vi "Velociprobe_Nanopositioner_Control_RT 2.vi"() -> ()   [LabVIEW 2015] (continued)
        n12 = invoke on="Waveform Graph 2" class="WFGraph (strict)" method="Reinit To Default"() -> (error out=w50:errorcluster)  [unwired: 3 in, 2 out]
        n13 = xnode "Read/Write Control"("FPGA VI Reference In"=w42, "error in"=w41) -> ("FPGA VI Reference Out"=w40:refnum<k20>, "error out"=w39:errorcluster, "error out (FPGA)"=w57:errorcluster)
        n14 = Merge Errors "Merge Errors"(w39, w57, w50) -> (w38:errorcluster)
      }
      frame "Update Controller Info" {
        w294 = dbl[] [1.0, 2.0, 4.0, 5.0]  # Index_soscoeff_zz1
        w133 = dbl[] [1.0, 2.0, 4.0, 5.0]  # Index_soscoeff_yz1
        w154 = dbl[] [1.0, 2.0, 4.0, 5.0]  # Index_soscoeff_xz1
        w185 = dbl[] [1.0, 2.0, 4.0, 5.0]  # Index_soscoeff_zy1
        w315 = dbl[] [1.0, 2.0, 4.0, 5.0]  # Index_soscoeff_yy1
        w206 = dbl[] [1.0, 2.0, 4.0, 5.0]  # Index_soscoeff_xy1
        w232 = dbl[] [1.0, 2.0, 4.0, 5.0]  # Index_soscoeff_zx1
        w341 = dbl[] [1.0, 2.0, 4.0, 5.0]  # Index_soscoeff_xx1
        w258 = dbl[] [1.0, 2.0, 4.0, 5.0]  # Index_soscoeff_yx1
        w114 = "%.10f"  # format (%.3f)
        w122 = "%.10f"  # format (%.3f)
        w135 = "%.10f"  # format (%.3f)
        w143 = "%.10f"  # format (%.3f)
        w166 = "%.10f"  # format (%.3f)
        w174 = "%.10f"  # format (%.3f)
        w187 = "%.10f"  # format (%.3f)
        w195 = "%.10f"  # format (%.3f)
        w213 = "%.10f"  # format (%.3f)
        w221 = "%.10f"  # format (%.3f)
        w239 = "%.10f"  # format (%.3f)
        w247 = "%.10f"  # format (%.3f)
        w275 = "%.10f"  # format (%.3f)
        w283 = "%.10f"  # format (%.3f)
        w296 = "%.10f"  # format (%.3f)
        w304 = "%.10f"  # format (%.3f)
        w105 = fxp<+/-,42,9> 0.0 ("fixed-point type")
        w317 = "%.10f"  # format (%.3f)
        w104 = fxp<+/-,64,9> 0.0 ("fixed-point type")
        w330 = "%.10f"  # format (%.3f)
        w348 = 40000000.0  # FPGA Clock Rate (Hz)
        w81 = 1
        n15 = local read "sos gain SF Controller yy1c"() -> (w269:fxp<+/-,42,9>)
        n16 = local read "sos gain SF Controller yz1c"() -> (w90:fxp<+/-,42,9>)
        n17 = local read "sos gain SF Controller yx1c"() -> (w236:fxp<+/-,42,9>)
        n18 = local read "sos gain SF Controller xy1c"() -> (w159:fxp<+/-,42,9>)
        n19 = local read "sos gain SF Controller zy1c"() -> (w164:fxp<+/-,42,9>)
        n20 = local read "sos gain SF Controller xz1c"() -> (w106:fxp<+/-,42,9>)
        n21 = local read "sos gain SF Controller xx1c"() -> (w319:fxp<+/-,42,9>)
        n22 = local read "sos gain SF Controller zz1c"() -> (w267:fxp<+/-,42,9>)
        n23 = local read "sos gain SF Controller zx1c"() -> (w211:fxp<+/-,42,9>)
        n24 = local read "-a01(2) yy1c"() -> (w273:fxp<+/-,64,9>[])
        n25 = local read "-a02(2) yy1c"() -> (w272:fxp<+/-,64,9>[])
        n26 = local read "-a01(2) yz1c"() -> (w111:fxp<+/-,64,9>[])
        n27 = local read "-a02(2) yz1c"() -> (w112:fxp<+/-,64,9>[])
        n28 = local read "-a01(2) yx1c"() -> (w237:fxp<+/-,64,9>[])
        n29 = local read "-a02(2) yx1c"() -> (w233:fxp<+/-,64,9>[])
        n30 = local read "-a01(2) xy1c"() -> (w155:fxp<+/-,64,9>[])
        n31 = local read "-a02(2) xy1c"() -> (w156:fxp<+/-,64,9>[])
        n32 = local read "-a01(2) zy1c"() -> (w160:fxp<+/-,64,9>[])
        n33 = local read "-a02(2) zy1c"() -> (w161:fxp<+/-,64,9>[])
        n34 = local read "-a01(2) xz1c"() -> (w110:fxp<+/-,64,9>[])
        n35 = local read "-a02(2) xz1c"() -> (w109:fxp<+/-,64,9>[])
        n36 = local read "-a01(2) xx1c"() -> (w328:fxp<+/-,64,9>[])
        n37 = local read "-a02(2) xx1c"() -> (w327:fxp<+/-,64,9>[])
        n38 = local read "-a01(2) zz1c"() -> (w268:fxp<+/-,64,9>[])
        n39 = local read "-a02(2) zz1c"() -> (w264:fxp<+/-,64,9>[])
        n40 = local read "-a01(2) zx1c"() -> (w207:fxp<+/-,64,9>[])
        n41 = local read "-a02(2) zx1c"() -> (w208:fxp<+/-,64,9>[])
        n42 = local read "b01(2) yy1c"() -> (w271:fxp<+/-,64,9>[])
        n43 = local read "b02(2) yy1c"() -> (w270:fxp<+/-,64,9>[])
        n44 = local read "b01(2) yz1c"() -> (w76:fxp<+/-,64,9>[])
        n45 = local read "b02(2) yz1c"() -> (w75:fxp<+/-,64,9>[])
        n46 = local read "b01(2) yx1c"() -> (w234:fxp<+/-,64,9>[])
        n47 = local read "b02(2) yx1c"() -> (w235:fxp<+/-,64,9>[])
        n48 = local read "b01(2) xy1c"() -> (w157:fxp<+/-,64,9>[])
        n49 = local read "b02(2) xy1c"() -> (w158:fxp<+/-,64,9>[])
        n50 = local read "b01(2) zy1c"() -> (w162:fxp<+/-,64,9>[])
        n51 = local read "b02(2) zy1c"() -> (w163:fxp<+/-,64,9>[])
        n52 = local read "b01(2) xz1c"() -> (w108:fxp<+/-,64,9>[])
        n53 = local read "b02(2) xz1c"() -> (w107:fxp<+/-,64,9>[])
        n54 = local read "b01(2) xx1c"() -> (w326:fxp<+/-,64,9>[])
        n55 = local read "b02(2) xx1c"() -> (w325:fxp<+/-,64,9>[])
        n56 = local read "b01(2) zz1c"() -> (w265:fxp<+/-,64,9>[])
        n57 = local read "b02(2) zz1c"() -> (w266:fxp<+/-,64,9>[])
        n58 = local read "b01(2) zx1c"() -> (w209:fxp<+/-,64,9>[])
        n59 = local read "b02(2) zx1c"() -> (w210:fxp<+/-,64,9>[])
        n60 = Or(x="Optics Z Reset", y="Reset All") -> (x .or. y?=w103:bool)
        n61 = Or(x="Sample Z Reset", y="Reset All") -> (x .or. y?=w100:bool)
        n62 = Or(x="Optics X Reset", y="Reset All") -> (x .or. y?=w262:bool)
        n63 = Or(x="Optics Y Reset", y="Reset All") -> (x .or. y?=w260:bool)
        n64 = Or(x="Sample X Reset", y="Reset All") -> (x .or. y?=w102:bool)
        n65 = Or(x="Sample Y Reset", y="Reset All") -> (x .or. y?=w101:bool)
        n66 = call-poly <vilib>:"Read Delimited Spreadsheet.vi"("file path (dialog if empty)"="file path soscoeff_xx1", "format (%.3f)"=w330) -> ("all rows"=w329:dbl[][])  [unwired: 8 in, 5 out]
        n67 = call-poly <vilib>:"Read Delimited Spreadsheet.vi"("file path (dialog if empty)"="file path soscoeff_zy1", "format (%.3f)"=w174) -> ("all rows"=w173:dbl[][])  [unwired: 8 in, 5 out]
        n68 = call-poly <vilib>:"Read Delimited Spreadsheet.vi"("file path (dialog if empty)"="file path soscoeff_xy1", "format (%.3f)"=w195) -> ("all rows"=w194:dbl[][])  [unwired: 8 in, 5 out]
        n69 = call-poly <vilib>:"Read Delimited Spreadsheet.vi"("file path (dialog if empty)"="file path soscoeff_zx1", "format (%.3f)"=w221) -> ("all rows"=w220:dbl[][])  [unwired: 8 in, 5 out]
        n70 = call-poly <vilib>:"Read Delimited Spreadsheet.vi"("file path (dialog if empty)"="file path soscoeff_xz1", "format (%.3f)"=w143) -> ("all rows"=w142:dbl[][])  [unwired: 8 in, 5 out]
        n71 = call-poly <vilib>:"Read Delimited Spreadsheet.vi"("file path (dialog if empty)"="file path soscoeff_yx1", "format (%.3f)"=w247) -> ("all rows"=w246:dbl[][])  [unwired: 8 in, 5 out]
        n72 = call-poly <vilib>:"Read Delimited Spreadsheet.vi"("file path (dialog if empty)"="file path soscoeff_yy1", "format (%.3f)"=w304) -> ("all rows"=w303:dbl[][])  [unwired: 8 in, 5 out]
        n73 = call-poly <vilib>:"Read Delimited Spreadsheet.vi"("file path (dialog if empty)"="file path soscoeff_yz1", "format (%.3f)"=w122) -> ("all rows"=w121:dbl[][])  [unwired: 8 in, 5 out]
        n74 = call-poly <vilib>:"Read Delimited Spreadsheet.vi"("file path (dialog if empty)"="file path soscoeff_zz1", "format (%.3f)"=w283) -> ("all rows"=w282:dbl[][])  [unwired: 8 in, 5 out]
        n75 = Transpose 2D Array(2D array=w329) -> (transposed array=w340:dbl[][])
        n76 = Transpose 2D Array(2D array=w173) -> (transposed array=w184:dbl[][])
        n77 = Transpose 2D Array(2D array=w194) -> (transposed array=w205:dbl[][])
        n78 = Transpose 2D Array(2D array=w220) -> (transposed array=w231:dbl[][])
        n79 = Transpose 2D Array(2D array=w142) -> (transposed array=w153:dbl[][])
        n80 = Transpose 2D Array(2D array=w246) -> (transposed array=w257:dbl[][])
        n81 = Transpose 2D Array(2D array=w303) -> (transposed array=w314:dbl[][])
        n82 = Transpose 2D Array(2D array=w121) -> (transposed array=w132:dbl[][])
        n83 = Transpose 2D Array(2D array=w282) -> (transposed array=w293:dbl[][])
        n84 = call-poly <vilib>:"Read Delimited Spreadsheet.vi"("file path (dialog if empty)"="file path sos gain SF Controller_xx1", "format (%.3f)"=w317) -> ("all rows"=w316:dbl[][])  [unwired: 8 in, 5 out]
        n85 = call-poly <vilib>:"Read Delimited Spreadsheet.vi"("file path (dialog if empty)"="file path sos gain SF Controller_zy1", "format (%.3f)"=w166) -> ("all rows"=w165:dbl[][])  [unwired: 8 in, 5 out]
        n86 = call-poly <vilib>:"Read Delimited Spreadsheet.vi"("file path (dialog if empty)"="file path sos gain SF Controller_xy1", "format (%.3f)"=w187) -> ("all rows"=w186:dbl[][])  [unwired: 8 in, 5 out]
        n87 = call-poly <vilib>:"Read Delimited Spreadsheet.vi"("file path (dialog if empty)"="file path sos gain SF Controller_zx1", "format (%.3f)"=w213) -> ("all rows"=w212:dbl[][])  [unwired: 8 in, 5 out]
        n88 = call-poly <vilib>:"Read Delimited Spreadsheet.vi"("file path (dialog if empty)"="file path sos gain SF Controller_xz1", "format (%.3f)"=w135) -> ("all rows"=w134:dbl[][])  [unwired: 8 in, 5 out]
        n89 = call-poly <vilib>:"Read Delimited Spreadsheet.vi"("file path (dialog if empty)"="file path sos gain SF Controller_yx1", "format (%.3f)"=w239) -> ("all rows"=w238:dbl[][])  [unwired: 8 in, 5 out]
        n90 = call-poly <vilib>:"Read Delimited Spreadsheet.vi"("file path (dialog if empty)"="file path sos gain SF Controller_yy1", "format (%.3f)"=w296) -> ("all rows"=w295:dbl[][])  [unwired: 8 in, 5 out]
        n91 = call-poly <vilib>:"Read Delimited Spreadsheet.vi"("file path (dialog if empty)"="file path sos gain SF Controller_yz1", "format (%.3f)"=w114) -> ("all rows"=w113:dbl[][])  [unwired: 8 in, 5 out]
        n92 = call-poly <vilib>:"Read Delimited Spreadsheet.vi"("file path (dialog if empty)"="file path sos gain SF Controller_zz1", "format (%.3f)"=w275) -> ("all rows"=w274:dbl[][])  [unwired: 8 in, 5 out]
        n93 = xnode "Read/Write Control"("FPGA VI Reference In"=w69, "error in"=w70, "Controller Time Period (uSec)"="Controller Time Period (uSec)", "Controller Output Time Period (uSec)"="Controller Output Time Period (uSec)", "System Loop Type"="System Loop Type", "Controller Output Upper Limit"="Controller Output Upper Limit", "Controller Output Lower Limit"="Controller Output Lower Limit", "X-Stage nm to V Scaling"="X-Stage nm to V Scaling", "X-Stage Scaling Direction"="X-Stage Scaling Direction", "Y-Stage nm to V Scaling"="Y-Stage nm to V Scaling", "Z-Stage nm to V Scaling"="Z-Stage nm to V Scaling", "Plant Output Time Period (uSec)"="Plant Output Time Period (uSec)", "Reset Optics X"=w262, "Reset Optics Y"=w260, "Reset Optics Z"=w103, "Reset Sample X"=w102, "Reset Sample Y"=w101, "Reset Sample Z"=w100, "Optics X Stage Resolution (nm)"="Optics X Stage Resolution (nm)", "Optics Y Stage Resolution (nm)"="Optics Y Stage Resolution (nm)", "Optics Z Stage Resolution (nm)"="Optics Z Stage Resolution (nm)", "Sample X Stage Resolution (nm)"="Sample X Stage Resolution (nm)", "Sample Y Stage Resolution (nm)"="Sample Y Stage Resolution (nm)", "Sample Z Stage Resolution (nm)"="Sample Z Stage Resolution (nm)", "Scaling mV to V"="Scaling mV to V", "-a01(2) xx1"=w328, "-a02(2) xx1"=w327, "b01(2) xx1"=w326, "b02(2) xx1"=w325, "sos gain SF Controller xx1"=w319, "-a01(2) yy1"=w273, "-a02(2) yy1"=w272, "b01(2) yy1"=w271, "b02(2) yy1"=w270, "sos gain SF Controller yy1"=w269, "-a01(2) zz1"=w268, "-a02(2) zz1"=w264, "b01(2) zz1"=w265, "b02(2) zz1"=w266, "sos gain SF Controller zz1"=w267, "-a01(2) yx1"=w237, "-a02(2) yx1"=w233, "b01(2) yx1"=w234, "b02(2) yx1"=w235, "sos gain SF Controller yx1"=w236, "-a01(2) zx1"=w207, "-a02(2) zx1"=w208, "b01(2) zx1"=w209, "b02(2) zx1"=w210, "sos gain SF Controller zx1"=w211, "-a01(2) xy1"=w155, "-a02(2) xy1"=w156, "b01(2) xy1"=w157, "b02(2) xy1"=w158, "sos gain SF Controller xy1"=w159, "-a01(2) zy1"=w160, "-a02(2) zy1"=w161, "b01(2) zy1"=w162, "b02(2) zy1"=w163, "sos gain SF Controller zy1"=w164, "-a01(2) xz1"=w110, "-a02(2) xz1"=w109, "b01(2) xz1"=w108, "b02(2) xz1"=w107, "sos gain SF Controller xz1"=w106, "-a01(2) yz1"=w111, "-a02(2) yz1"=w112, "b01(2) yz1"=w76, "b02(2) yz1"=w75, "sos gain SF Controller yz1"=w90, "Analog Input Time Period (uSec)"="Analog Input Time Period (uSec)", "Optics and or Sample Stage"="Optics and or Sample Stage", "Y-Stage Scaling Direction"="Y-Stage Scaling Direction", "Z-Stage Scaling Direction"="Z-Stage Scaling Direction") -> ("FPGA VI Reference Out"=w68:refnum<k20>, "error out"=w67:errorcluster)
        n94 = for {
          tunnel: w341 -> [w517] mode=indexing
          tunnel: w340 -> [w516]
          tunnel: [w515] -> _ mode=indexing
          shift-right: [w515] -> w332
          shift-left: _ -> [w514]
          shift-left: _ -> [w513]
          shift-left: _ -> [w512]
          tunnel: [w514] -> w333
          tunnel: [w513] -> w334
          tunnel: [w512] -> w335
          n95 = Index Array "Index Array"(array=w516, index (row)=w517) -> (element=w515:dbl[])  [unwired: 1 in]
        }
        n96 = Index Array(array=w316, index (row)=0 ("index (row) 6")) -> (element=w324:dbl[])  [unwired: 1 in]
        n97 = for {
          tunnel: w185 -> [w415] mode=indexing
          tunnel: w184 -> [w414]
          tunnel: [w413] -> _ mode=indexing
          shift-right: [w413] -> w176
          shift-left: _ -> [w412]
          shift-left: _ -> [w411]
          shift-left: _ -> [w410]
          tunnel: [w412] -> w177
          tunnel: [w411] -> w178
          tunnel: [w410] -> w179
          n98 = Index Array "Index Array"(array=w414, index (row)=w415) -> (element=w413:dbl[])  [unwired: 1 in]
        }
        n99 = Index Array(array=w165, index (row)=0 ("index (row) 18")) -> (element=w172:dbl[])  [unwired: 1 in]
        n100 = for {
          tunnel: w206 -> [w432] mode=indexing
          tunnel: w205 -> [w431]
          tunnel: [w430] -> _ mode=indexing
          shift-right: [w430] -> w197
          shift-left: _ -> [w429]
          shift-left: _ -> [w428]
          shift-left: _ -> [w427]
          tunnel: [w429] -> w198
          tunnel: [w428] -> w199
          tunnel: [w427] -> w200
          n101 = Index Array "Index Array"(array=w431, index (row)=w432) -> (element=w430:dbl[])  [unwired: 1 in]
        }
        n102 = Index Array(array=w186, index (row)=0 ("index (row) 16")) -> (element=w193:dbl[])  [unwired: 1 in]
        n103 = for {
          tunnel: w232 -> [w449] mode=indexing
          tunnel: w231 -> [w448]
          tunnel: [w447] -> _ mode=indexing
          shift-right: [w447] -> w223
          shift-left: _ -> [w446]
          shift-left: _ -> [w445]
          shift-left: _ -> [w444]
          tunnel: [w446] -> w224
          tunnel: [w445] -> w225
          tunnel: [w444] -> w226
          n104 = Index Array "Index Array"(array=w448, index (row)=w449) -> (element=w447:dbl[])  [unwired: 1 in]
        }
        n105 = Index Array(array=w212, index (row)=0 ("index (row) 14")) -> (element=w219:dbl[])  [unwired: 1 in]
        n106 = for {
          tunnel: w154 -> [w398] mode=indexing
          tunnel: w153 -> [w397]
          tunnel: [w396] -> _ mode=indexing
          shift-right: [w396] -> w145
          shift-left: _ -> [w395]
          shift-left: _ -> [w394]
          shift-left: _ -> [w393]
          tunnel: [w395] -> w146
          tunnel: [w394] -> w147
          tunnel: [w393] -> w148
          n107 = Index Array "Index Array"(array=w397, index (row)=w398) -> (element=w396:dbl[])  [unwired: 1 in]
        }
        n108 = Index Array(array=w134, index (row)=0 ("index (row) 20")) -> (element=w141:dbl[])  [unwired: 1 in]
        n109 = for {
          tunnel: w258 -> [w466] mode=indexing
          tunnel: w257 -> [w465]
          tunnel: [w464] -> _ mode=indexing
          shift-right: [w464] -> w249
          shift-left: _ -> [w463]
          shift-left: _ -> [w462]
          shift-left: _ -> [w461]
          tunnel: [w463] -> w250
          tunnel: [w462] -> w251
          tunnel: [w461] -> w252
          n110 = Index Array "Index Array"(array=w465, index (row)=w466) -> (element=w464:dbl[])  [unwired: 1 in]
        }
        n111 = Index Array(array=w238, index (row)=0 ("index (row) 12")) -> (element=w245:dbl[])  [unwired: 1 in]
        n112 = for {
          tunnel: w315 -> [w500] mode=indexing
          tunnel: w314 -> [w499]
          tunnel: [w498] -> _ mode=indexing
          shift-right: [w498] -> w306
          shift-left: _ -> [w497]
          shift-left: _ -> [w496]
          shift-left: _ -> [w495]
          tunnel: [w497] -> w307
          tunnel: [w496] -> w308
          tunnel: [w495] -> w309
          n113 = Index Array "Index Array"(array=w499, index (row)=w500) -> (element=w498:dbl[])  [unwired: 1 in]
        }
        n114 = Index Array(array=w295, index (row)=0 ("index (row) 8")) -> (element=w302:dbl[])  [unwired: 1 in]
        n115 = for {
          tunnel: w133 -> [w381] mode=indexing
          tunnel: w132 -> [w380]
          tunnel: [w379] -> _ mode=indexing
          shift-right: [w379] -> w124
          shift-left: _ -> [w378]
          shift-left: _ -> [w377]
          shift-left: _ -> [w376]
          tunnel: [w378] -> w125
          tunnel: [w377] -> w126
          tunnel: [w376] -> w127
          n116 = Index Array "Index Array"(array=w380, index (row)=w381) -> (element=w379:dbl[])  [unwired: 1 in]
        }
        n117 = Index Array(array=w113, index (row)=0 ("index (row) 22")) -> (element=w120:dbl[])  [unwired: 1 in]
        n118 = Index Array(array=w274, index (row)=0 ("index (row) 10")) -> (element=w281:dbl[])  [unwired: 1 in]
        n119 = for {
          tunnel: w294 -> [w483] mode=indexing
          tunnel: w293 -> [w482]
          tunnel: [w481] -> _ mode=indexing
          shift-right: [w481] -> w285
          shift-left: _ -> [w480]
          shift-left: _ -> [w479]
          shift-left: _ -> [w478]
          tunnel: [w480] -> w286
          tunnel: [w479] -> w287
          tunnel: [w478] -> w288
          n120 = Index Array "Index Array"(array=w482, index (row)=w483) -> (element=w481:dbl[])  [unwired: 1 in]
        }
        n121 = Index Array(array=w324, index=0 ("index (row) 7")) -> (element=w322:dbl)
        n122 = Index Array(array=w172, index=0 ("index (row) 19")) -> (element=w170:dbl)
        n123 = Index Array(array=w193, index=0 ("index (row) 17")) -> (element=w191:dbl)
        n124 = Index Array(array=w219, index=0 ("index (row) 15")) -> (element=w217:dbl)
        n125 = Index Array(array=w141, index=0 ("index (row) 21")) -> (element=w139:dbl)
        n126 = Index Array(array=w245, index=0 ("index (row) 13")) -> (element=w243:dbl)
        n127 = Index Array(array=w302, index=0 ("index (row) 9")) -> (element=w300:dbl)
        n128 = Index Array(array=w120, index=0 ("index (row) 23")) -> (element=w118:dbl)
        n129 = Index Array(array=w281, index=0 ("index (row) 11")) -> (element=w279:dbl)
        n130 = xnode "Read/Write Control"("FPGA VI Reference In"=w68, "error in"=w67) -> ("FPGA VI Reference Out"=w66:refnum<k20>, "error out"=w65:errorcluster, "PI X-Stage Input (V)"=→"PI X-Stage Input (V)":fxp<+/-,20,5>, "PI Y-Stage Input (V)"=→"PI Y-Stage Input (V)":fxp<+/-,20,5>, "PI Z-Stage Input (V)"=→"PI Z-Stage Input (V)":fxp<+/-,20,5>, "X-Stage Input In Range?"=→"X-Stage Input In Range?":bool, "Y-Stage Input In Range?"=→"Y-Stage Input In Range?":bool, "Z-Stage Input In Range?"=→"Z-Stage Input In Range?":bool, "Measured Controller Time Period (Ticks)"=w349:u32, "Measured Controller Output Time Period (Ticks)"=w346:u32, "Measured Plant Output Time Period (Ticks)"=w82:u32, "Measured Analog Input Time Period (Ticks)"=→"Measured Analog Input Time Period (Ticks)":u32)
        "Measured Controller Time Period (Ticks)" <- w349
        "Measured Controller Output Time Period (Ticks)" <- w346
        "Measured Plant Output Time Period (Ticks)" <- w82
        n131 = To Fixed-Point(fixed-point type=w105, number=w191) -> (fixed-point=→"sos gain SF Controller xy1c":fxp<+/-,42,9>)
        n132 = To Fixed-Point(fixed-point type=w105, number=w300) -> (fixed-point=→"sos gain SF Controller yy1c":fxp<+/-,42,9>)
        n133 = To Fixed-Point(fixed-point type=w105, number=w170) -> (fixed-point=→"sos gain SF Controller zy1c":fxp<+/-,42,9>)
        n134 = To Fixed-Point(fixed-point type=w105, number=w139) -> (fixed-point=→"sos gain SF Controller xz1c":fxp<+/-,42,9>)
        n135 = To Fixed-Point(fixed-point type=w105, number=w118) -> (fixed-point=→"sos gain SF Controller yz1c":fxp<+/-,42,9>)
        n136 = To Fixed-Point(fixed-point type=w105, number=w243) -> (fixed-point=→"sos gain SF Controller yx1c":fxp<+/-,42,9>)
        n137 = To Fixed-Point(fixed-point type=w105, number=w217) -> (fixed-point=→"sos gain SF Controller zx1c":fxp<+/-,42,9>)
        n138 = To Fixed-Point(fixed-point type=w105, number=w279) -> (fixed-point=→"sos gain SF Controller zz1c":fxp<+/-,42,9>)
        n139 = To Fixed-Point(fixed-point type=w105, number=w322) -> (fixed-point=→"sos gain SF Controller xx1c":fxp<+/-,42,9>)
        n140 = Divide(x=w81, y=w348) -> (x/y=w83:dbl)
        n141 = Multiply(x=w83, y=w349) -> (x*y=w350:dbl)
        "Measured Controller Loop Rate (secs)" <- w350
        n142 = Multiply(x=w83, y=w346) -> (x*y=w358:dbl)
        "Measured Controller Output Loop Rate (secs)" <- w358
        n143 = Multiply(x=w83, y=w82) -> (x*y=w354:dbl)
        "Measured Plant Output Loop Rate (secs)" <- w354
        n144 = Multiply(x=w83, y=w82) -> (x*y=w87:dbl)
        "Measured Analog Input Loop Rate (secs)" <- w87
        n145 = for {
          tunnel: w177 -> [w426] mode=indexing
          tunnel: [w425] -> w183 mode=indexing
          tunnel: w176 -> [w424] mode=indexing
          tunnel: w179 -> [w423] mode=indexing
          tunnel: w178 -> [w422] mode=indexing
          tunnel: [w421] -> w182 mode=indexing
          tunnel: [w420] -> w181 mode=indexing
          tunnel: [w419] -> w180 mode=indexing
          tunnel: w104 -> [w416]
          n146 = Negate(x=w426) -> (-x=w418:dbl)
          n147 = Negate(x=w424) -> (-x=w417:dbl)
          n148 = To Fixed-Point(fixed-point type=w416, number=w418) -> (fixed-point=w425:fxp<+/-,64,9>)
          n149 = To Fixed-Point(fixed-point type=w416, number=w417) -> (fixed-point=w421:fxp<+/-,64,9>)
          n150 = To Fixed-Point(fixed-point type=w416, number=w423) -> (fixed-point=w420:fxp<+/-,64,9>)
          n151 = To Fixed-Point(fixed-point type=w416, number=w422) -> (fixed-point=w419:fxp<+/-,64,9>)
        }
        "-a01(2) zy1c" <- w183
        "-a02(2) zy1c" <- w182
        "b01(2) zy1c" <- w181
        "b02(2) zy1c" <- w180
        n152 = for {
          tunnel: w333 -> [w528] mode=indexing
          tunnel: [w527] -> w339 mode=indexing
          tunnel: w332 -> [w526] mode=indexing
          tunnel: w335 -> [w525] mode=indexing
          tunnel: w334 -> [w524] mode=indexing
          tunnel: [w523] -> w338 mode=indexing
          tunnel: [w522] -> w337 mode=indexing
          tunnel: [w521] -> w336 mode=indexing
          tunnel: w104 -> [w518]
          n153 = Negate(x=w528) -> (-x=w520:dbl)
          n154 = Negate(x=w526) -> (-x=w519:dbl)
          n155 = To Fixed-Point(fixed-point type=w518, number=w520) -> (fixed-point=w527:fxp<+/-,64,9>)
          n156 = To Fixed-Point(fixed-point type=w518, number=w519) -> (fixed-point=w523:fxp<+/-,64,9>)
          n157 = To Fixed-Point(fixed-point type=w518, number=w525) -> (fixed-point=w522:fxp<+/-,64,9>)
          n158 = To Fixed-Point(fixed-point type=w518, number=w524) -> (fixed-point=w521:fxp<+/-,64,9>)
        }
        "-a01(2) xx1c" <- w339
        "-a02(2) xx1c" <- w338
        "b01(2) xx1c" <- w337
        "b02(2) xx1c" <- w336
        n159 = for {
          tunnel: w198 -> [w443] mode=indexing
          tunnel: [w442] -> w204 mode=indexing
          tunnel: w197 -> [w441] mode=indexing
          tunnel: w200 -> [w440] mode=indexing
          tunnel: w199 -> [w439] mode=indexing
          tunnel: [w438] -> w203 mode=indexing
          tunnel: [w437] -> w202 mode=indexing
          tunnel: [w436] -> w201 mode=indexing
          tunnel: w104 -> [w433]
          n160 = Negate(x=w443) -> (-x=w435:dbl)
          n161 = Negate(x=w441) -> (-x=w434:dbl)
          n162 = To Fixed-Point(fixed-point type=w433, number=w435) -> (fixed-point=w442:fxp<+/-,64,9>)
          n163 = To Fixed-Point(fixed-point type=w433, number=w434) -> (fixed-point=w438:fxp<+/-,64,9>)
          n164 = To Fixed-Point(fixed-point type=w433, number=w440) -> (fixed-point=w437:fxp<+/-,64,9>)
          n165 = To Fixed-Point(fixed-point type=w433, number=w439) -> (fixed-point=w436:fxp<+/-,64,9>)
        }
        "-a01(2) xy1c" <- w204
        "-a02(2) xy1c" <- w203
        "b01(2) xy1c" <- w202
        "b02(2) xy1c" <- w201
        n166 = for {
          tunnel: w146 -> [w409] mode=indexing
          tunnel: [w408] -> w152 mode=indexing
          tunnel: w145 -> [w407] mode=indexing
          tunnel: w148 -> [w406] mode=indexing
          tunnel: w147 -> [w405] mode=indexing
          tunnel: [w404] -> w151 mode=indexing
          tunnel: [w403] -> w150 mode=indexing
          tunnel: [w402] -> w149 mode=indexing
          tunnel: w104 -> [w399]
          n167 = Negate(x=w409) -> (-x=w401:dbl)
          n168 = Negate(x=w407) -> (-x=w400:dbl)
          n169 = To Fixed-Point(fixed-point type=w399, number=w401) -> (fixed-point=w408:fxp<+/-,64,9>)
          n170 = To Fixed-Point(fixed-point type=w399, number=w400) -> (fixed-point=w404:fxp<+/-,64,9>)
          n171 = To Fixed-Point(fixed-point type=w399, number=w406) -> (fixed-point=w403:fxp<+/-,64,9>)
          n172 = To Fixed-Point(fixed-point type=w399, number=w405) -> (fixed-point=w402:fxp<+/-,64,9>)
        }
        "-a01(2) xz1c" <- w152
        "-a02(2) xz1c" <- w151
        "b01(2) xz1c" <- w150
        "b02(2) xz1c" <- w149
        n173 = for {
          tunnel: w307 -> [w511] mode=indexing
          tunnel: [w510] -> w313 mode=indexing
          tunnel: w306 -> [w509] mode=indexing
          tunnel: w309 -> [w508] mode=indexing
          tunnel: w308 -> [w507] mode=indexing
          tunnel: [w506] -> w312 mode=indexing
          tunnel: [w505] -> w311 mode=indexing
          tunnel: [w504] -> w310 mode=indexing
          tunnel: w104 -> [w501]
          n174 = Negate(x=w511) -> (-x=w503:dbl)
          n175 = Negate(x=w509) -> (-x=w502:dbl)
          n176 = To Fixed-Point(fixed-point type=w501, number=w503) -> (fixed-point=w510:fxp<+/-,64,9>)
          n177 = To Fixed-Point(fixed-point type=w501, number=w502) -> (fixed-point=w506:fxp<+/-,64,9>)
          n178 = To Fixed-Point(fixed-point type=w501, number=w508) -> (fixed-point=w505:fxp<+/-,64,9>)
          n179 = To Fixed-Point(fixed-point type=w501, number=w507) -> (fixed-point=w504:fxp<+/-,64,9>)
        }
        "-a01(2) yy1c" <- w313
        "-a02(2) yy1c" <- w312
        "b01(2) yy1c" <- w311
        "b02(2) yy1c" <- w310
        n180 = for {
          tunnel: w224 -> [w460] mode=indexing
          tunnel: [w459] -> w230 mode=indexing
          tunnel: w223 -> [w458] mode=indexing
          tunnel: w226 -> [w457] mode=indexing
          tunnel: w225 -> [w456] mode=indexing
          tunnel: [w455] -> w229 mode=indexing
          tunnel: [w454] -> w228 mode=indexing
          tunnel: [w453] -> w227 mode=indexing
          tunnel: w104 -> [w450]
          n181 = Negate(x=w460) -> (-x=w452:dbl)
          n182 = Negate(x=w458) -> (-x=w451:dbl)
          n183 = To Fixed-Point(fixed-point type=w450, number=w452) -> (fixed-point=w459:fxp<+/-,64,9>)
          n184 = To Fixed-Point(fixed-point type=w450, number=w451) -> (fixed-point=w455:fxp<+/-,64,9>)
          n185 = To Fixed-Point(fixed-point type=w450, number=w457) -> (fixed-point=w454:fxp<+/-,64,9>)
          n186 = To Fixed-Point(fixed-point type=w450, number=w456) -> (fixed-point=w453:fxp<+/-,64,9>)
        }
        "-a01(2) zx1c" <- w230
        "-a02(2) zx1c" <- w229
        "b01(2) zx1c" <- w228
        "b02(2) zx1c" <- w227
        n187 = for {
          tunnel: w250 -> [w477] mode=indexing
          tunnel: [w476] -> w256 mode=indexing
          tunnel: w249 -> [w475] mode=indexing
          tunnel: w252 -> [w474] mode=indexing
          tunnel: w251 -> [w473] mode=indexing
          tunnel: [w472] -> w255 mode=indexing
          tunnel: [w471] -> w254 mode=indexing
          tunnel: [w470] -> w253 mode=indexing
          tunnel: w104 -> [w467]
          n188 = Negate(x=w477) -> (-x=w469:dbl)
          n189 = Negate(x=w475) -> (-x=w468:dbl)
          n190 = To Fixed-Point(fixed-point type=w467, number=w469) -> (fixed-point=w476:fxp<+/-,64,9>)
          n191 = To Fixed-Point(fixed-point type=w467, number=w468) -> (fixed-point=w472:fxp<+/-,64,9>)
          n192 = To Fixed-Point(fixed-point type=w467, number=w474) -> (fixed-point=w471:fxp<+/-,64,9>)
          n193 = To Fixed-Point(fixed-point type=w467, number=w473) -> (fixed-point=w470:fxp<+/-,64,9>)
        }
        "-a01(2) yx1c" <- w256
        "-a02(2) yx1c" <- w255
        "b01(2) yx1c" <- w254
        "b02(2) yx1c" <- w253
        n194 = for {
          tunnel: w125 -> [w392] mode=indexing
          tunnel: [w391] -> w131 mode=indexing
          tunnel: w124 -> [w390] mode=indexing
          tunnel: w127 -> [w389] mode=indexing
          tunnel: w126 -> [w388] mode=indexing
          tunnel: [w387] -> w130 mode=indexing
          tunnel: [w386] -> w129 mode=indexing
          tunnel: [w385] -> w128 mode=indexing
          tunnel: w104 -> [w382]
          n195 = Negate(x=w392) -> (-x=w384:dbl)
          n196 = Negate(x=w390) -> (-x=w383:dbl)
          n197 = To Fixed-Point(fixed-point type=w382, number=w384) -> (fixed-point=w391:fxp<+/-,64,9>)
          n198 = To Fixed-Point(fixed-point type=w382, number=w383) -> (fixed-point=w387:fxp<+/-,64,9>)
          n199 = To Fixed-Point(fixed-point type=w382, number=w389) -> (fixed-point=w386:fxp<+/-,64,9>)
          n200 = To Fixed-Point(fixed-point type=w382, number=w388) -> (fixed-point=w385:fxp<+/-,64,9>)
        }
        "-a01(2) yz1c" <- w131
        "-a02(2) yz1c" <- w130
        "b01(2) yz1c" <- w129
        "b02(2) yz1c" <- w128
        n201 = Divide(x=w81, y=w350) -> (x/y=w361:dbl)
        n202 = Divide(x=w81, y=w358) -> (x/y=w357:dbl)
        n203 = Divide(x=w81, y=w354) -> (x/y=w353:dbl)
        n204 = for {
          tunnel: w286 -> [w494] mode=indexing
          tunnel: [w493] -> w292 mode=indexing
          tunnel: w285 -> [w492] mode=indexing
          tunnel: w288 -> [w491] mode=indexing
          tunnel: w287 -> [w490] mode=indexing
          tunnel: [w489] -> w291 mode=indexing
          tunnel: [w488] -> w290 mode=indexing
          tunnel: [w487] -> w289 mode=indexing
          tunnel: w104 -> [w484]
          n205 = Negate(x=w494) -> (-x=w486:dbl)
          n206 = Negate(x=w492) -> (-x=w485:dbl)
          n207 = To Fixed-Point(fixed-point type=w484, number=w486) -> (fixed-point=w493:fxp<+/-,64,9>)
          n208 = To Fixed-Point(fixed-point type=w484, number=w485) -> (fixed-point=w489:fxp<+/-,64,9>)
          n209 = To Fixed-Point(fixed-point type=w484, number=w491) -> (fixed-point=w488:fxp<+/-,64,9>)
          n210 = To Fixed-Point(fixed-point type=w484, number=w490) -> (fixed-point=w487:fxp<+/-,64,9>)
        }
        "-a01(2) zz1c" <- w292
        "-a02(2) zz1c" <- w291
        "b01(2) zz1c" <- w290
        "b02(2) zz1c" <- w289
        n211 = Divide(x=w81, y=w87) -> (x/y=w86:dbl)
        n212 = Divide(x=w361, y=1000) -> (x/y=→"Measured Controller Loop Rate (kHz)":dbl)
        n213 = Divide(x=w357, y=1000) -> (x/y=→"Measured Controller Output Loop Rate (kHz)":dbl)
        n214 = Divide(x=w353, y=1000) -> (x/y=→"Measured Plant Output Loop Rate (kHz)":dbl)
        n215 = Divide(x=w86, y=1000) -> (x/y=→"Measured Analog Input Loop Rate (kHz)":dbl)
      }
      frame "Update Reference Info" {
        w606 = 40000000.0  # FPGA Clock Rate (Hz)
        w600 = 1
        w613 = 40000000.0  # FPGA Clock Rate (Hz)
        w607 = 1
        w618 = errorcluster {"status"=FALSE, "code"=0, "source"=""}  # error in (no error)
        w621 = errorcluster {"status"=FALSE, "code"=0, "source"=""}  # error in (no error)
        w635 = 40000000.0  # FPGA Clock Rate (Hz)
        w629 = 1
        w647 = errorcluster {"status"=FALSE, "code"=0, "source"=""}  # error in (no error)
        w614 = 40000000.0  # FPGA clock rate (Hz)
        n216 = case shown="\"EPICS Snake Scan\"" "Snake Scan Reference FPGA or EPICS" {
          tunnel: ["X Ramp Start (nm)" w665] -> w547
          tunnel: ["X Ramp End (nm)" w664] -> w546
          tunnel: ["Fly Scan Start" w670] -> w545
          tunnel: ["Y Ramp Start (nm)" w663] -> w544
          tunnel: ["Y Ramp End (nm)" w662] -> w543
          tunnel: ["Y Vertical Step Size (nm)" w666] -> w542
          tunnel: ["X Horizontal Step Size (nm)" w669] -> w541
          tunnel: [w656 w667] -> w540
          tunnel: ["Y Vertical Step Size (nm)" w666] -> w533
          tunnel: ["X Ramp Start (nm)" w665] -> w532
          tunnel: ["X Ramp End (nm)" w664] -> w531
          tunnel: ["Y Ramp Start (nm)" w663] -> w530
          tunnel: ["Y Ramp End (nm)" w662] -> w529
          frame "FPGA Snake Scan", Default {
            n217 = local read "DT Frequency (Hz)"() -> (w656:dbl)
          }
          frame "EPICS Snake Scan" {
            w668 = fxp<+/-,16,16> 0.0 ("fixed-point type")
            n218 = shared-variable "RT CompactRIO Target\\RT_EPICS_Shared_Variables.lvlib\\2iddVELO:VP:Trigger_Freq_Hz"() -> (w667:dbl)  [unwired: 1 in, 1 out]
            "2iddVELO:VP:Trigger_Freq_Hz" <- w667
            n219 = shared-variable "RT CompactRIO Target\\RT_EPICS_Shared_Variables.lvlib\\2iddVELO:VP:Y_Step_Size_nm"() -> (w672:dbl)  [unwired: 1 in, 1 out]
            "2iddVELO:VP:Y_Step_Size_nm" <- w672
            n220 = shared-variable "RT CompactRIO Target\\RT_EPICS_Shared_Variables.lvlib\\2iddVELO:VP:X_Step_Size_nm"() -> (w671:dbl)  [unwired: 1 in, 1 out]
            "2iddVELO:VP:X_Step_Size_nm" <- w671
            n221 = shared-variable "RT CompactRIO Target\\RT_EPICS_Shared_Variables.lvlib\\2iddVELO:VP:Y_Start_nm"() -> (w673:dbl)  [unwired: 1 in, 1 out]
            n222 = shared-variable "RT CompactRIO Target\\RT_EPICS_Shared_Variables.lvlib\\2iddVELO:VP:Y_End_nm"() -> (w661:dbl)  [unwired: 1 in, 1 out]
            n223 = shared-variable "RT CompactRIO Target\\RT_EPICS_Shared_Variables.lvlib\\2iddVELO:VP:Flyscan_Start"() -> (w670:bool)  [unwired: 1 in, 1 out]
            "2iddVELO:VP:Flyscan_Start" <- w670
            n224 = shared-variable "RT CompactRIO Target\\RT_EPICS_Shared_Variables.lvlib\\2iddVELO:VP:X_Start_nm"() -> (w675:dbl)  [unwired: 1 in, 1 out]
            "2iddVELO:VP:X_Start_nm" <- w675
            n225 = shared-variable "RT CompactRIO Target\\RT_EPICS_Shared_Variables.lvlib\\2iddVELO:VP:X_End_nm"() -> (w674:dbl)  [unwired: 1 in, 1 out]
            "2iddVELO:VP:X_End_nm" <- w674
            n226 = Negate(x=w661) -> (-x=w660:dbl)
            "2iddVELO:VP:Y_End_nm" <- w660
            n227 = Negate(x=w673) -> (-x=w659:dbl)
            "2iddVELO:VP:Y_Start_nm" <- w659
            n228 = To Fixed-Point(fixed-point type=w668, number=w675) -> (fixed-point=w665:fxp<+/-,16,16>)
            n229 = To Fixed-Point(fixed-point type=w668, number=w674) -> (fixed-point=w664:fxp<+/-,16,16>)
            n230 = To Fixed-Point(fixed-point type=w668, number=w659) -> (fixed-point=w663:fxp<+/-,16,16>)
            n231 = To Fixed-Point(fixed-point type=w668, number=w660) -> (fixed-point=w662:fxp<+/-,16,16>)
            n232 = To Fixed-Point(fixed-point type=w668, number=w672) -> (fixed-point=w666:fxp<+/-,16,16>)
            n233 = To Fixed-Point(fixed-point type=w668, number=w671) -> (fixed-point=w669:fxp<+/-,16,16>)
          }
        }
        n234 = local read "X Ramp Period (usec)"() -> (w549:fxp<+,24,24>)
        n235 = local read "Y Ramp Period (usec)"() -> (w550:fxp<+,24,24>)
        n236 = case shown="\"Sawtooth Wave\"" "Z Reference Wave Selection" {
          tunnel: "Z frequency (Hz)" -> [w676 w677 w679 w681 w682]
          tunnel: [w676 w677 w678 w681 w682] -> w575
          tunnel: w574 -> [_ _ w680 _ _]
          frame "Constant", Default {
          }
          frame "Sine Wave" {
          }
          frame "Sawtooth Wave" {
            n237 = Multiply(x=w680, y=w679) -> (x*y=w678:dbl)
          }
          frame "Square Wave" {
          }
          frame "Filtered White Noise" {
          }
        }
        n238 = case shown="\"Custom Ramp Wave\"" "Y Reference Wave Selection" {
          tunnel: "Y frequency (Hz)" -> [w683 w684 w685 w686]
          tunnel: [w683 w684 w685 w686] -> w580
          tunnel: w577 -> [_ _ _ _]
          frame "Constant", Default {
          }
          frame "Sine Wave" {
          }
          frame "Custom Ramp Wave" {
          }
          frame "Filtered White Noise" {
          }
        }
        n239 = case shown="\"Custom Up Down Ramp\"" "X Reference Wave Selection" {
          tunnel: "X frequency (Hz)" -> [w687 w688 w689 w690]
          tunnel: [w687 w688 w689 w690] -> w584
          tunnel: w582 -> [_ _ _ _]
          frame "Constant", Default {
          }
          frame "Sine Wave" {
          }
          frame "Custom Up Down Ramp" {
          }
          frame "Filtered White Noise" {
          }
        }
        n240 = call <vilib>:"Normalize Signal Generation Parameters.vi"("frequency (Hz)"=w580, "FPGA clock rate (Hz)"=w614, "phase offset (deg)"="Y phase offset (deg)", "error in (no error)"=w621) -> ("frequency (periods/tick)"=w617:fxp<+,32,0>, "phase offset (periods)"=w616:fxp<+,32,0>, "error out"=→"error out (Sig Gen) 2":errorcluster)  [unwired: 6 in, 3 out]
        "Y frequency (periods/tick)" <- w617
        "Y phase offset (periods)" <- w616
        n241 = call <vilib>:"Normalize Signal Generation Parameters.vi"("frequency (Hz)"=w575, "FPGA clock rate (Hz)"=w614, "phase offset (deg)"="Z phase offset (deg)", "error in (no error)"=w618) -> ("frequency (periods/tick)"=w615:fxp<+,32,0>, "phase offset (periods)"=w593:fxp<+,32,0>, "error out"=→"error out (Sig Gen) 3":errorcluster)  [unwired: 6 in, 3 out]
        "Z frequency (periods/tick)" <- w615
        "Z phase offset (periods)" <- w593
        n242 = call <vilib>:"Normalize Signal Generation Parameters.vi"("frequency (Hz)"=w584, "FPGA clock rate (Hz)"=w614, "phase offset (deg)"="X phase offset (deg)", "error in (no error)"=w647) -> ("frequency (periods/tick)"=w646:fxp<+,32,0>, "phase offset (periods)"=w624:fxp<+,32,0>, "error out"=→"error out (Sig Gen)":errorcluster)  [unwired: 6 in, 3 out]
        "X frequency (periods/tick)" <- w646
        "X phase offset (periods)" <- w624
        n243 = xnode "Read/Write Control"("FPGA VI Reference In"=w539, "error in"=w538, "X Reference Time Period (uSec)"="X Reference Time Period (uSec)", "Y Reference Time Period (uSec)"="Y Reference Time Period (uSec)", "Z Reference Time Period (uSec)"="Z Reference Time Period (uSec)", "X Reference Wave Selection"="X Reference Wave Selection", "Y Reference Wave Selection"="Y Reference Wave Selection", "Z Reference Wave Selection"="Z Reference Wave Selection", "X Reference Reset"="X Reference Reset", "Y Reference Reset"="Y Reference Reset", "Z Reference Reset"="Z Reference Reset", "X Reference Amplitude (nm)"="X Reference Amplitude (nm)", "Y Reference Amplitude (nm)"="Y Reference Amplitude (nm)", "Z Reference Amplitude (nm)"="Z Reference Amplitude (nm)", "X Frequency (periods/tick)"=w646, "X Phase Offset (periods)"=w624, "Y Frequency (periods/tick)"=w617, "Y Phase Offset (periods)"=w616, "Z Frequency (periods/tick)"=w615, "Z Phase Offset (periods)"=w593, "X Reference DC Offset (nm)"="X Reference DC Offset (nm)", "Y Reference DC Offset (nm)"="Y Reference DC Offset (nm)", "Z Reference DC Offset (nm)"="Z Reference DC Offset (nm)", "X White Noise Amplitude"="X White Noise Amplitude", "X White Noise Seed"="X White Noise Seed", "Y White Noise Amplitude"="Y White Noise Amplitude", "Y White Noise Seed"="Y White Noise Seed", "Z White Noise Amplitude"="Z White Noise Amplitude", "Z White Noise Seed"="Z White Noise Seed", "Mod 3 AI0 V to nm Scaling"="Mod 3 AI0 V to nm Scaling", "Mod 3 AI1 V to nm Scaling"="Mod 3 AI1 V to nm Scaling", "Mod 3 AI2 V to nm Scaling"="Mod 3 AI2 V to nm Scaling", "X Ramp Period (usec)"=w549, "X Ramp Start (nm)"=w547, "X Ramp End (nm)"=w546, "X Start Marker (nm)"="X Start Marker (nm)", "Fly Scan Start"=w545, "Y Ramp Period (usec)"=w550, "Y Ramp Start (nm)"=w544, "Y Ramp End (nm)"=w543, "Y Ramp Drop Size (nm)"=w542, "Y Start Marker (nm)"="Y Start Marker (nm)") -> ("FPGA VI Reference Out"=w537:refnum<k20>, "error out"=w536:errorcluster)